vi "Super Market Billing System Edited 1.1.vi"() -> ()   [LabVIEW 2021]
uses:
  <vilib>/Utility/file.llb/Write Delimited Spreadsheet (string).vi
  <vilib>/regexp/Match Regular Expression.xnode
panel:
  in  "Tab Control":enum32{"Page 1", "Page 2", "Page 3"}(tab)
  out "Horizontal Progress Bar":u8(slide) scale=0.0..100.0
  in  "Password":string
  in  "Cashier User Name":string
  in  "OK Button":bool
  in  "Rice 5kg":bool
  in  "Dal 1kg":bool
  in  "Salt 400g":bool
  in  "Coconut Oil 1L":bool
  in  "Chilli Powder 100g":bool
  in  "Curry Powder 100g":bool
  in  "Turmeric Powder 50g":bool
  in  "Milk Powder 1kg":bool
  in  "Sugar  1kg":bool
  out "Rs.":dbl
  out "Rs.":dbl
  out "Rs.":dbl
  out "Rs.":dbl
  in  "Quantitiy":dbl min=0.0 format="%#.1f"
  out "Rs.":dbl
  in  "Quantitiy":dbl min=0.0 format="%#.1f"
  out "Rs":dbl
  in  "Quantitiy":dbl min=0.0 format="%#.1f"
  out "Rs.":dbl
  in  "Quantitiy":dbl min=0.0 format="%#.1f"
  in  "Quantitiy":dbl min=0.0 format="%#.1f"
  in  "Quantitiy":dbl min=0.0 format="%#.1f"
  in  "Quantitiy":dbl min=0.0 format="%#.1f"
  in  "Quantitiy":dbl min=0.0 format="%#.1f"
  in  "Tea 100g":bool
  in  "Quantitiy":dbl min=0.0 format="%#.1f"
  in  "Quantitiy":dbl min=0.0 format="%#.1f"
  out "Rs.":dbl
  out "Rs.":dbl
  out "Rs.":dbl
  out "Rs.":dbl
  out "Rs.":dbl
  out "Rs.":dbl
  out "Rs.":dbl
  out "Rs. 5":dbl
  out "Rs. 6":dbl
  out "Rs.":dbl
  out "Rs.":dbl
  out "Rs.":dbl
  out "Rs.":dbl
  out "Discount   Rs.":dbl format="%#.2f"
  in  "kg":dbl min=0.0 format="%#.3f"
  in  "Papaya":bool
  in  "kg":dbl min=0.0 format="%#.3f"
  in  "Graps":bool
  in  "kg":dbl min=0.0 format="%#.3f"
  in  "Orange":bool
  in  "kg":dbl min=0.0 format="%#.3f"
  in  "Apple":bool
  in  "kg":dbl min=0.0 format="%#.3f"
  in  "Banana":bool
  out "Bill   Rs.":dbl format="%#.2f"
  out "Discount percentage":string
  out "Total Bill   Rs.":dbl format="%#.2f"
  in  "kg":dbl min=0.0 format="%#.3f"
  in  "Cabege":bool
  in  "kg":dbl min=0.0 format="%#.3f"
  in  "Bringle":bool
  in  "kg":dbl min=0.0 format="%#.3f"
  in  "Beans":bool
  in  "kg":dbl min=0.0 format="%#.3f"
  in  "Leeks":bool
  in  "kg":dbl min=0.0 format="%#.3f"
  in  "Carrot":bool
  in  "stop":bool
  in  "stop 2":bool
  out "Bill Details":string
  in  "stop 3":bool
  # "WELCOME   TO  ABC                  SUPERMARCKET.."
  # "Price per 1kg (Rs.)"
  # "Quantities(kg)"
  # "Price  (Rs.)"
  # "Quantities"
  # "Fruits"
  # "Product List"
  # "Vegetables"
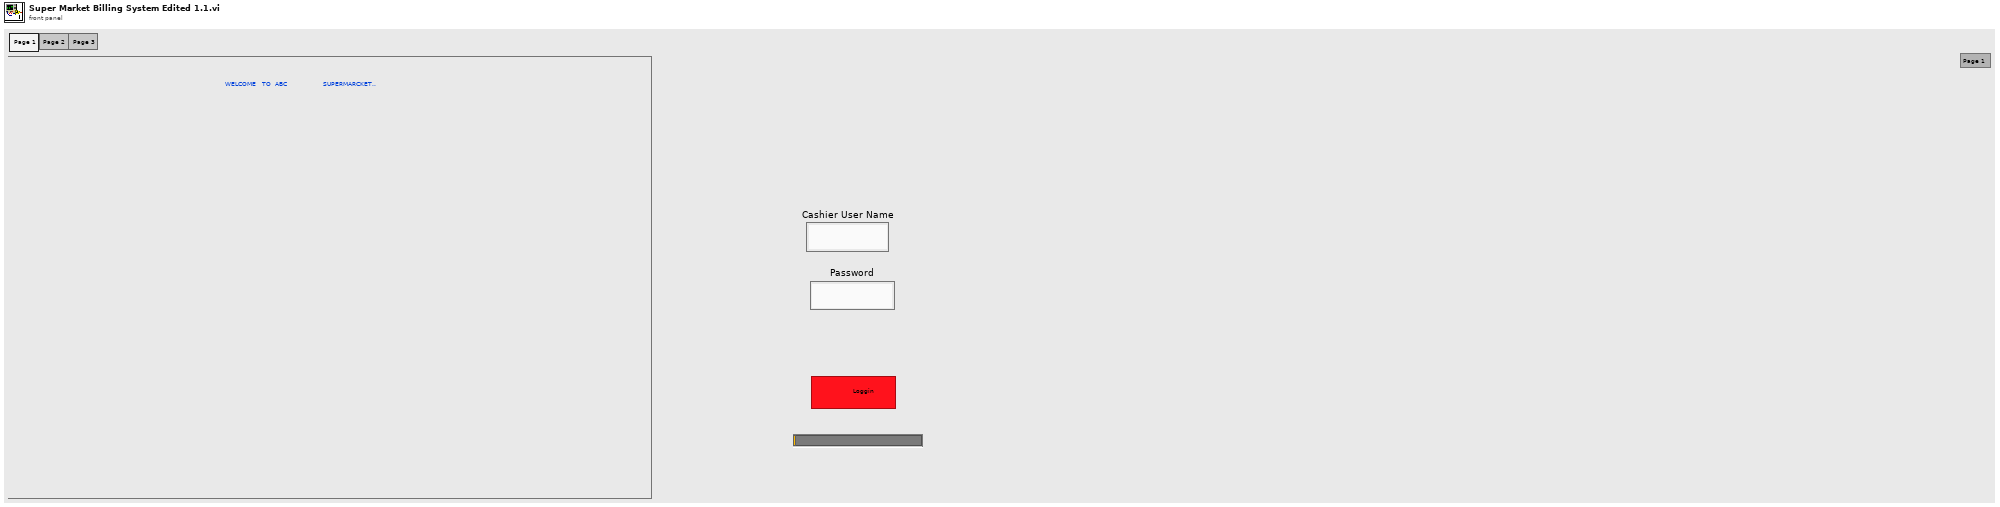
[diagram p1: front panel]
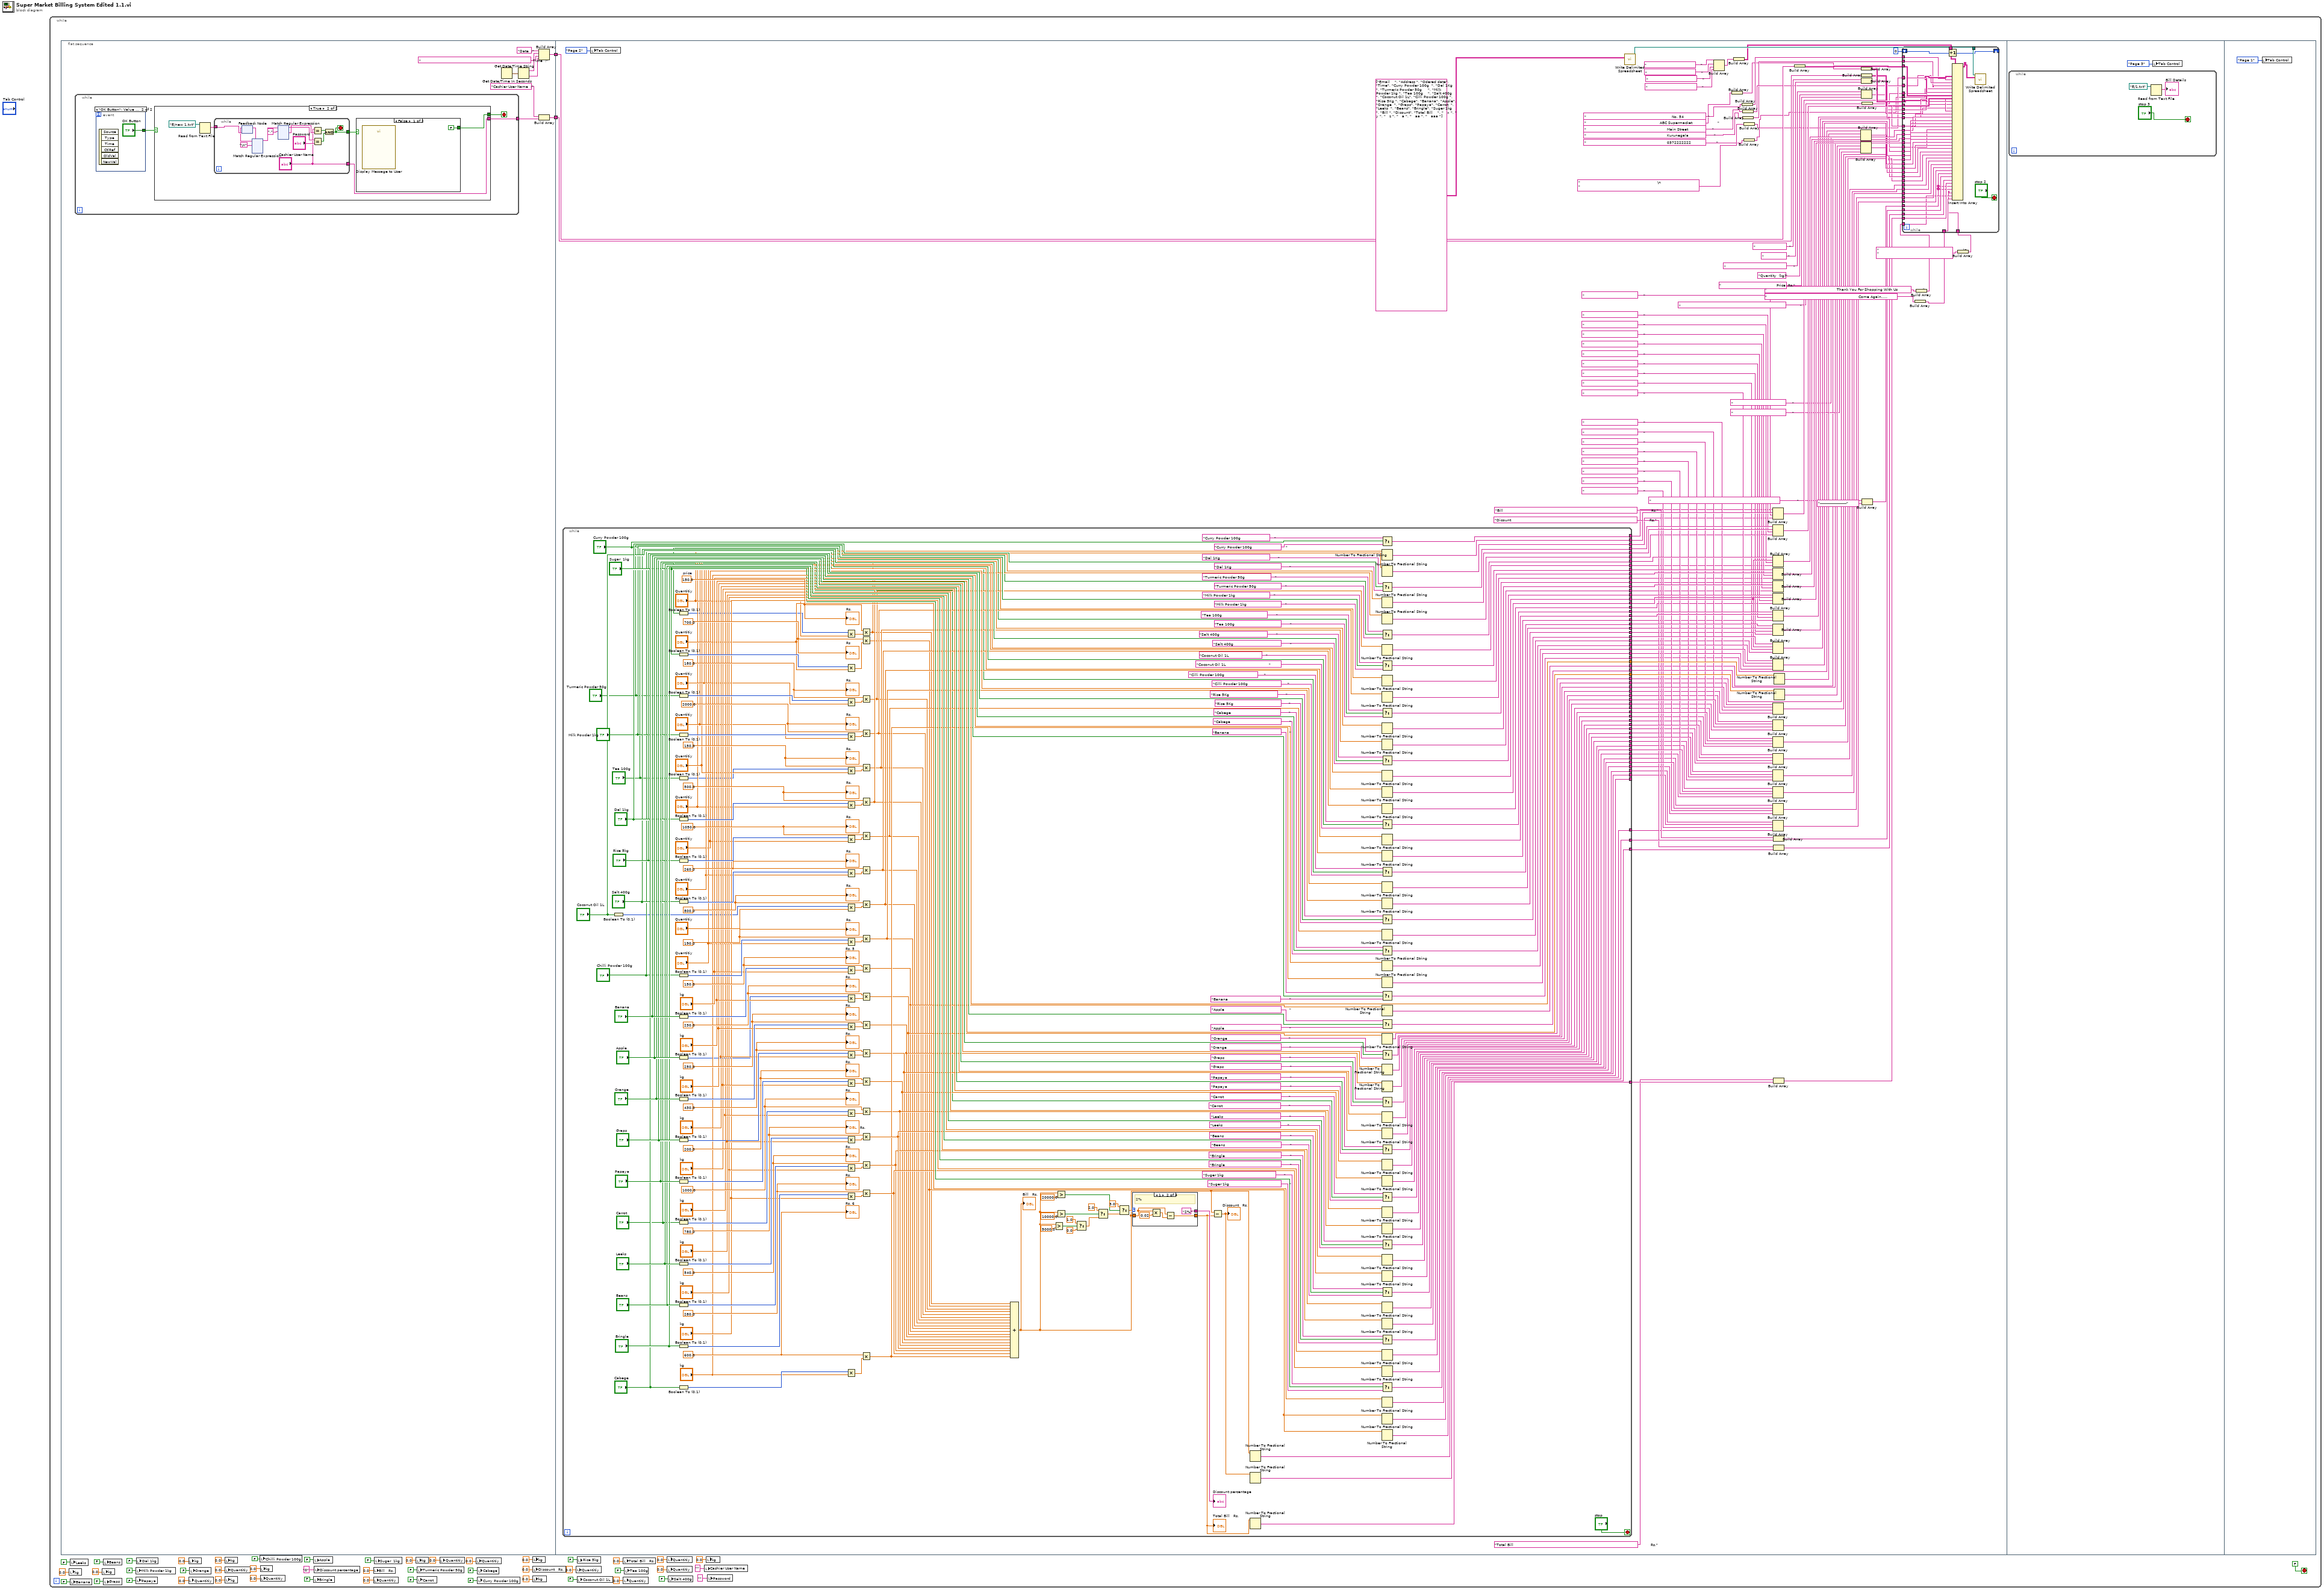
[diagram p0: block diagram]
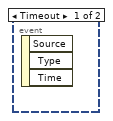
[diagram p2: hidden frame]
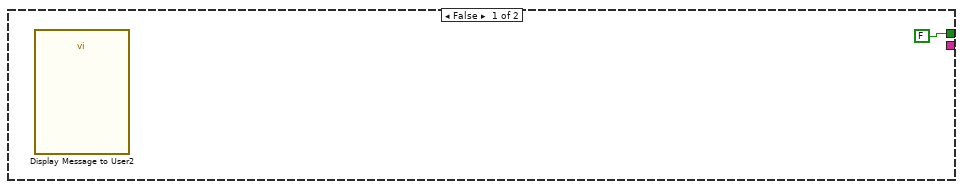
[diagram p3: hidden frame]
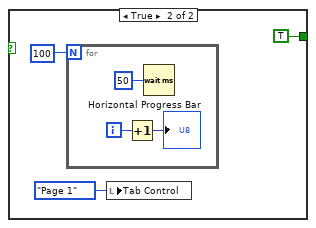
[diagram p4: hidden frame]
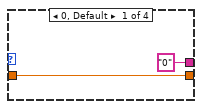
[diagram p5: hidden frame]
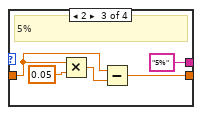
[diagram p6: hidden frame]
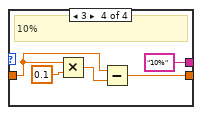
[diagram p7: hidden frame]
diagram:
  n1 = while {
    stop <- FALSE stop-if-true
    n2 = flat-sequence {
      tunnel: [w56] -> w48
      tunnel: [w52] -> w4
      tunnel: w48 -> [w351]
      tunnel: w4 -> [w418]
      frame #0 {
        n3 = while {
          tunnel: [w61] -> w50
          stop <- w60 stop-if-true
          n4 = event shown="[1] \"OK Button\": Value Change" {
            selector: _ -> [_ _]
            dyn-events: _ -> [_ _]
            timeout: _ -> [_ _]
            tunnel: [_ "OK Button"] -> w59
            event Timeout {
              n5 = event-data() -> ()  [unwired: 1 in, 3 out]
            }
            event "OK Button": Value Change {
              n6 = event-data() -> ()  [unwired: 1 in, 6 out]
            }
          }
          n7 = case shown="True" w59 {
            tunnel: [_ w66] -> w61
            tunnel: [FALSE w65] -> w60
            frame False {
              n8 = call "Display Message to User2"() -> ()  [unwired: 10 in, 2 out]
            }
            frame True {
              n9 = Read from Text File(file (use dialog)=path "E:/new 1.txt") -> (text=w68:string)  [unwired: 3 in, 3 out]
              n10 = while {
                tunnel: w68 -> [w88]
                tunnel: ["Cashier User Name"] -> w66
                tunnel: [w76] -> w64
                stop <- w76 stop-if-true
                n11 = feedback #1(w88) -> (w87:string)
                n12 = xnode "Match Regular Expression"("input string"=w87, "regular expression"="\n") -> ("before match"=w84:string, "after match"=w86:string)  [unwired: 4 in, 3 out]
                n13 = feedback-in #1(w86) -> ()
                n14 = xnode "Match Regular Expression"("input string"=w84, "regular expression"=",") -> ("before match"=w81:string, "after match"=w82:string)  [unwired: 4 in, 3 out]
                n15 = Equal?(x="Cashier User Name", y=w81) -> (x = y?=w79:bool)
                n16 = Equal?(x=w82, y="Password") -> (x = y?=w78:bool)
                n17 = And(x=w79, y=w78) -> (x .and. y?=w76:bool)
              }
              n18 = case shown="False" w64 {
                tunnel: [FALSE TRUE] -> w65
                frame False {
                  n19 = call "Display Message to User"() -> ()  [unwired: 10 in, 2 out]
                }
                frame True {
                  n20 = for {
                    N: 100 -> [_]
                    i -> [w73]
                    n21 = Increment(x=w73) -> (x+1=→"Horizontal Progress Bar":i32)
                    n22 = Wait (ms)(milliseconds to wait=u32 50 ("millisecond timer value")) -> ()  [unwired: 1 out]
                  }
                  n23 = local write "Tab Control"(enum32{"Page 1", "Page 2"}."Page 1" ("Tab Control")) -> ()
                }
              }
            }
          }
        }
        n24 = Get Date/Time In Seconds() -> (seconds since 1Jan1904=w57:timestamp)
        n25 = Get Date/Time String(seconds (now)=w57) -> (date string=w55:string, time string=w58:string)  [unwired: 2 in]
        n26 = Build Array("Date  :" ("element"), w55, "                                                                                             Time  :" ("element"), w58) -> (w56:string[])
        n27 = Build Array("Cashier User Name  :" ("element"), w50) -> (w52:string[])
      }
      frame #1 {
        n28 = while {
          tunnel: [w693] -> w471
          tunnel: [w690] -> w473
          tunnel: [w689] -> w474
          tunnel: [w681] -> w387
          tunnel: [w661] -> w441
          tunnel: [w660] -> w361
          tunnel: [w652] -> w357
          tunnel: [w651] -> w356
          tunnel: [w650] -> w355
          tunnel: [w649] -> w354
          tunnel: [w648] -> w358
          tunnel: [w647] -> w359
          tunnel: [w646] -> w432
          tunnel: ["kg"] -> w477
          tunnel: ["kg"] -> w476
          tunnel: [w642] -> w439
          tunnel: [w640] -> w438
          tunnel: [w637] -> w437
          tunnel: [w636] -> w436
          tunnel: [w635] -> w435
          tunnel: [w632] -> w434
          tunnel: [w629] -> w433
          tunnel: [w628] -> w431
          tunnel: [w601] -> w360
          tunnel: [w600] -> w333
          tunnel: [w599] -> w469
          tunnel: [w598] -> w468
          tunnel: [w597] -> w374
          tunnel: [w596] -> w465
          tunnel: [w595] -> w458
          tunnel: [w594] -> w462
          tunnel: [w593] -> w460
          tunnel: [w524] -> w459
          tunnel: [w590] -> w470
          tunnel: [w575] -> w407
          tunnel: [w588] -> w456
          tunnel: [w586] -> w467
          tunnel: [w584] -> w466
          tunnel: [w579] -> w464
          tunnel: [w522] -> w463
          tunnel: [w578] -> w461
          tunnel: [w577] -> w457
          tunnel: [w574] -> w406
          tunnel: [w573] -> w404
          tunnel: [w552] -> w402
          tunnel: [w551] -> w400
          tunnel: [w550] -> w398
          tunnel: [w548] -> w396
          tunnel: [w547] -> w394
          tunnel: [w536] -> w392
          tunnel: [w546] -> w390
          tunnel: [w545] -> w388
          tunnel: [w535] -> w385
          tunnel: [w544] -> w383
          tunnel: [w543] -> w380
          tunnel: [w542] -> w379
          tunnel: [w531] -> w377
          tunnel: [w541] -> w375
          tunnel: [w530] -> w372
          tunnel: [w540] -> w370
          tunnel: [w539] -> w368
          tunnel: [w538] -> w366
          tunnel: [w537] -> _
          stop <- "stop" stop-if-true
          w705 = 200.0 ("price")
          w702 = 430.0 ("price")
          w699 = 250.0 ("price")
          w697 = 230.0 ("price")
          w694 = 150.0 ("price")
          w720 = 600.0 ("price")
          w717 = 280.0 ("price")
          w714 = 540.0 ("price")
          w711 = 780.0 ("price")
          w708 = 1000.0 ("price")
          w747 = 150.0 ("price")
          w745 = 700.0 ("price")
          w742 = 2000.0 ("price")
          w739 = 180.0 ("price")
          w736 = 150.0  # price
          w759 = 190.0 ("price")
          w757 = 800.0 ("price")
          w754 = 260.0 ("price")
          w752 = 500.0 ("price")
          w749 = 1050.0 ("price")
          n29 = Boolean To (0,1)(Boolean="Coconut Oil 1L") -> (0, 1=w532:i16)
          n30 = Boolean To (0,1)(Boolean="Curry Powder 100g") -> (0, 1=w525:i16)
          n31 = Boolean To (0,1)(Boolean="Sugar  1kg") -> (0, 1=w746:i16)
          n32 = Boolean To (0,1)(Boolean="Turmeric Powder 50g") -> (0, 1=w740:i16)
          n33 = Boolean To (0,1)(Boolean="Milk Powder 1kg") -> (0, 1=w741:i16)
          n34 = Boolean To (0,1)(Boolean="Tea 100g") -> (0, 1=w528:i16)
          n35 = Boolean To (0,1)(Boolean="Dal 1kg") -> (0, 1=w686:i16)
          n36 = Boolean To (0,1)(Boolean="Rice 5kg") -> (0, 1=w688:i16)
          n37 = Boolean To (0,1)(Boolean="Salt 400g") -> (0, 1=w753:i16)
          n38 = Boolean To (0,1)(Boolean="Chilli Powder 100g") -> (0, 1=w687:i16)
          n39 = Boolean To (0,1)(Boolean="Banana") -> (0, 1=w685:i16)
          n40 = Boolean To (0,1)(Boolean="Apple") -> (0, 1=w534:i16)
          n41 = Boolean To (0,1)(Boolean="Orange") -> (0, 1=w698:i16)
          n42 = Boolean To (0,1)(Boolean="Graps") -> (0, 1=w703:i16)
          n43 = Boolean To (0,1)(Boolean="Papaya") -> (0, 1=w704:i16)
          n44 = Boolean To (0,1)(Boolean="Carrot") -> (0, 1=w707:i16)
          n45 = Boolean To (0,1)(Boolean="Leeks") -> (0, 1=w712:i16)
          n46 = Boolean To (0,1)(Boolean="Beans") -> (0, 1=w713:i16)
          n47 = Boolean To (0,1)(Boolean="Bringle") -> (0, 1=w718:i16)
          n48 = Boolean To (0,1)(Boolean="Cabege") -> (0, 1=w719:i16)
          n49 = Multiply(x=w525, y="Quantitiy") -> (x*y=w737:dbl)
          n50 = Multiply(x=w746, y="Quantitiy") -> (x*y=w744:dbl)
          n51 = Multiply(x=w740, y="Quantitiy") -> (x*y=w738:dbl)
          n52 = Multiply(x=w741, y="Quantitiy") -> (x*y=w743:dbl)
          n53 = Multiply(x=w528, y="Quantitiy") -> (x*y=w748:dbl)
          n54 = Multiply(x=w686, y="Quantitiy") -> (x*y=w751:dbl)
          n55 = Multiply(x=w688, y="Quantitiy") -> (x*y=w750:dbl)
          n56 = Multiply(x=w753, y="Quantitiy") -> (x*y=w755:dbl)
          n57 = Multiply(x=w532, y="Quantitiy") -> (x*y=w756:dbl)
          n58 = Multiply(x=w687, y="Quantitiy") -> (x*y=w760:dbl)
          n59 = Multiply(x=w685, y="kg") -> (x*y=w695:dbl)
          n60 = Multiply(x=w534, y="kg") -> (x*y=w696:dbl)
          n61 = Multiply(x=w698, y="kg") -> (x*y=w700:dbl)
          n62 = Multiply(x=w703, y="kg") -> (x*y=w701:dbl)
          n63 = Multiply(x=w704, y="kg") -> (x*y=w706:dbl)
          n64 = Multiply(x=w707, y="kg") -> (x*y=w709:dbl)
          n65 = Multiply(x=w712, y="kg") -> (x*y=w710:dbl)
          n66 = Multiply(x=w713, y="kg") -> (x*y=w715:dbl)
          n67 = Multiply(x=w718, y="kg") -> (x*y=w716:dbl)
          n68 = Multiply(x=w719, y="kg") -> (x*y=w721:dbl)
          n69 = Multiply(x=w736, y=w737) -> (x*y=w526:dbl)
          n70 = Multiply(x=w745, y=w744) -> (x*y=w553:dbl)
          n71 = Multiply(x=w739, y=w738) -> (x*y=w555:dbl)
          n72 = Multiply(x=w742, y=w743) -> (x*y=w556:dbl)
          n73 = Multiply(x=w747, y=w748) -> (x*y=w557:dbl)
          n74 = Multiply(x=w752, y=w751) -> (x*y=w559:dbl)
          n75 = Multiply(x=w749, y=w750) -> (x*y=w558:dbl)
          n76 = Multiply(x=w754, y=w755) -> (x*y=w560:dbl)
          n77 = Multiply(x=w757, y=w756) -> (x*y=w561:dbl)
          n78 = Multiply(x=w759, y=w760) -> (x*y=w562:dbl)
          n79 = Multiply(x=w694, y=w695) -> (x*y=w563:dbl)
          n80 = Multiply(x=w697, y=w696) -> (x*y=w564:dbl)
          n81 = Multiply(x=w699, y=w700) -> (x*y=w565:dbl)
          n82 = Multiply(x=w702, y=w701) -> (x*y=w566:dbl)
          n83 = Multiply(x=w705, y=w706) -> (x*y=w567:dbl)
          n84 = Multiply(x=w708, y=w709) -> (x*y=w568:dbl)
          n85 = Multiply(x=w711, y=w710) -> (x*y=w571:dbl)
          n86 = Multiply(x=w714, y=w715) -> (x*y=w570:dbl)
          n87 = Multiply(x=w717, y=w716) -> (x*y=w572:dbl)
          n88 = Multiply(x=w720, y=w721) -> (x*y=w569:dbl)
          n89 = Compound Arithmetic op=ADD(w526, w553, w555, w556, w557, w559, w558, w560, w561, w562, w563, w564, w565, w566, w567, w568, w571, w570, w572, w569) -> (w554:dbl)
          "Bill   Rs." <- w554
          n90 = Greater?(x=w554, y=5000.0) -> (0:w733:bool)
          n91 = Greater?(x=w554, y=20000.0) -> (0:w735:bool)
          n92 = Greater?(x=w554, y=10000.0) -> (0:w734:bool)
          n93 = Select(t=1.0, s=w733, f=0.0) -> (s? t:f=w729:dbl)
          n94 = Select(t=2.0, s=w734, f=w729) -> (s? t:f=w730:dbl)
          n95 = Select(t=3.0, s=w735, f=w730) -> (s? t:f=w731:dbl)
          n96 = case shown="1" w731 {
            tunnel: [w762 w766 w769 w774] -> w692
            tunnel: w554 -> [w762 w765 w770 w775]
            tunnel: ["0" ("discount") "2%" ("discount") "5%" ("discount") "10%" ("discount")] -> w732
            frame 0, Default {
            }
            frame 1 {
              # "2%"
              n97 = Multiply(x=w765, y=0.02) -> (x*y=w763:dbl)
              n98 = Subtract(x=w765, y=w763) -> (x-y=w766:dbl)
            }
            frame 2 {
              # "5%"
              n99 = Multiply(x=w770, y=0.05) -> (x*y=w771:dbl)
              n100 = Subtract(x=w770, y=w771) -> (x-y=w769:dbl)
            }
            frame 3 {
              # "10%"
              n101 = Multiply(x=w775, y=0.1) -> (x*y=w776:dbl)
              n102 = Subtract(x=w775, y=w776) -> (x-y=w774:dbl)
            }
          }
          "Total Bill   Rs." <- w692
          "Discount percentage" <- w732
          n103 = Subtract(x=w554, y=w692) -> (x-y=w691:dbl)
          "Discount   Rs." <- w691
          n104 = Number To Fractional String(number=w554) -> (F-format string=w693:string)  [unwired: 3 in]
          n105 = Number To Fractional String(number=w691) -> (F-format string=w689:string)  [unwired: 3 in]
          n106 = Number To Fractional String(number=w692) -> (F-format string=w690:string)  [unwired: 3 in]
          n107 = Select(t="Curry Powder 100g                            ", s="Curry Powder 100g", f="Curry Powder 100g                            ") -> (s? t:f=w600:string)
          n108 = Number To Fractional String(number="Quantitiy") -> (F-format string=w590:string)  [unwired: 3 in]
          n109 = Number To Fractional String(number=w526) -> (F-format string=w538:string)  [unwired: 3 in]
          n110 = Select(t="Dal 1Kg                                                ", s="Dal 1kg", f="Dal 1Kg                                                ") -> (s? t:f=w524:string)
          n111 = Number To Fractional String(number="Quantitiy") -> (F-format string=w577:string)  [unwired: 3 in]
          n112 = Number To Fractional String(number=w559) -> (F-format string=w531:string)  [unwired: 3 in]
          n113 = Select(t="Turmeric Powder 50g                         ", s="Turmeric Powder 50g", f="Turmeric Powder 50g                        ") -> (s? t:f=w599:string)
          n114 = Number To Fractional String(number=w555) -> (F-format string=w539:string)  [unwired: 3 in]
          n115 = Select(t="Milk Powder 1kg                                ", s="Milk Powder 1kg", f="Milk Powder 1kg                                ") -> (s? t:f=w598:string)
          n116 = Number To Fractional String(number="Quantitiy") -> (F-format string=w586:string)  [unwired: 3 in]
          n117 = Number To Fractional String(number=w556) -> (F-format string=w540:string)  [unwired: 3 in]
          n118 = Select(t="Tea 100g                                             ", s="Tea 100g", f="Tea 100g                                              ") -> (s? t:f=w597:string)
          n119 = Number To Fractional String(number="Quantitiy") -> (F-format string=w584:string)  [unwired: 3 in]
          n120 = Number To Fractional String(number=w557) -> (F-format string=w530:string)  [unwired: 3 in]
          n121 = Select(t="Salt 400g                                               ", s="Salt 400g", f="Salt 400g                                               ") -> (s? t:f=w596:string)
          n122 = Number To Fractional String(number="Quantitiy") -> (F-format string=w588:string)  [unwired: 3 in]
          n123 = Number To Fractional String(number="Quantitiy") -> (F-format string=w579:string)  [unwired: 3 in]
          n124 = Number To Fractional String(number=w560) -> (F-format string=w542:string)  [unwired: 3 in]
          n125 = Select(t="Coconut Oil 1L                               ", s="Coconut Oil 1L", f="Coconut Oil 1L                                    ") -> (s? t:f=w595:string)
          n126 = Number To Fractional String(number="Quantitiy") -> (F-format string=w522:string)  [unwired: 3 in]
          n127 = Number To Fractional String(number=w561) -> (F-format string=w543:string)  [unwired: 3 in]
          n128 = Select(t="Cilli Powder 100g                                 ", s="Chilli Powder 100g", f="Cilli Powder 100g                                 ") -> (s? t:f=w594:string)
          n129 = Number To Fractional String(number="Quantitiy") -> (F-format string=w578:string)  [unwired: 3 in]
          n130 = Number To Fractional String(number=w562) -> (F-format string=w544:string)  [unwired: 3 in]
          n131 = Select(t="Rise 5Kg                                               ", s="Rice 5kg", f="Rise 5Kg                                              ") -> (s? t:f=w593:string)
          n132 = Number To Fractional String(number=w558) -> (F-format string=w541:string)  [unwired: 3 in]
          n133 = Select(t="Cabege                                                ", s="Cabege", f="Cabege                                                 ") -> (s? t:f=w646:string)
          n134 = Number To Fractional String(number="kg") -> (F-format string=w628:string)  [unwired: 3 in]
          n135 = Number To Fractional String(number=w569) -> (F-format string=w552:string)  [unwired: 3 in]
          n136 = Select(t="Banana                                                  ", s="Banana", f="Banana                                                   ") -> (s? t:f=w681:string)
          n137 = Number To Fractional String(number=w563) -> (F-format string=w535:string)  [unwired: 3 in]
          n138 = Select(t="Apple                                                      ", s="Apple", f="Apple                                                      ") -> (s? t:f=w661:string)
          n139 = Number To Fractional String(number=w564) -> (F-format string=w545:string)  [unwired: 3 in]
          n140 = Select(t="Orange                                                   ", s="Orange", f="Orange                                                    ") -> (s? t:f=w660:string)
          n141 = Number To Fractional String(number="kg") -> (F-format string=w642:string)  [unwired: 3 in]
          n142 = Number To Fractional String(number=w565) -> (F-format string=w546:string)  [unwired: 3 in]
          n143 = Select(t="Graps                                                      " ("f"), s="Graps", f="Graps                                                       ") -> (s? t:f=w652:string)
          n144 = Number To Fractional String(number="kg") -> (F-format string=w640:string)  [unwired: 3 in]
          n145 = Number To Fractional String(number=w566) -> (F-format string=w536:string)  [unwired: 3 in]
          n146 = Select(t="Papaya                                                    ", s="Papaya", f="Papaya                                                    ") -> (s? t:f=w651:string)
          n147 = Number To Fractional String(number="kg") -> (F-format string=w637:string)  [unwired: 3 in]
          n148 = Number To Fractional String(number=w567) -> (F-format string=w547:string)  [unwired: 3 in]
          n149 = Select(t="Carrot                                                      ", s="Carrot", f="Carrot                                                       ") -> (s? t:f=w650:string)
          n150 = Number To Fractional String(number="kg") -> (F-format string=w636:string)  [unwired: 3 in]
          n151 = Number To Fractional String(number=w568) -> (F-format string=w548:string)  [unwired: 3 in]
          n152 = Select(t="Leeks                                                       ", s="Leeks", f="Leeks                                                      ") -> (s? t:f=w649:string)
          n153 = Number To Fractional String(number="kg") -> (F-format string=w635:string)  [unwired: 3 in]
          n154 = Number To Fractional String(number=w571) -> (F-format string=w550:string)  [unwired: 3 in]
          n155 = Select(t="Beans                                                       ", s="Beans", f="Beans                                                      ") -> (s? t:f=w648:string)
          n156 = Number To Fractional String(number="kg") -> (F-format string=w632:string)  [unwired: 3 in]
          n157 = Number To Fractional String(number=w570) -> (F-format string=w551:string)  [unwired: 3 in]
          n158 = Select(t="Bringle                                                      ", s="Bringle", f="Bringle                                                      ") -> (s? t:f=w647:string)
          n159 = Number To Fractional String(number="kg") -> (F-format string=w629:string)  [unwired: 3 in]
          n160 = Number To Fractional String(number=w572) -> (F-format string=w573:string)  [unwired: 3 in]
          n161 = Select(t="Suger 1kg                                                  ", s="Sugar  1kg", f="Suger 1kg                                                  ") -> (s? t:f=w601:string)
          n162 = Number To Fractional String(number="Quantitiy") -> (F-format string=w575:string)  [unwired: 3 in]
          n163 = Number To Fractional String(number=w553) -> (F-format string=w537:string)  [unwired: 3 in]
          n164 = Number To Fractional String(number=w553) -> (F-format string=w574:string)  [unwired: 3 in]
          "Rs." <- w749
          "Rs." <- w752
          "Rs." <- w754
          "Rs." <- w757
          "Rs." <- w759
          "Rs." <- w736
          "Rs." <- w739
          "Rs." <- w742
          "Rs" <- w745
          "Rs." <- w747
          "Rs." <- w708
          "Rs." <- w711
          "Rs." <- w714
          "Rs." <- w717
          "Rs. 6" <- w720
          "Rs. 5" <- w694
          "Rs." <- w697
          "Rs." <- w699
          "Rs." <- w702
          "Rs." <- w705
        }
        n165 = local write "Tab Control"(enum32{"Page 1", "Page 2"}."Page 2" ("Tab Control")) -> ()
        n166 = call-poly <vilib>:"Write Delimited Spreadsheet.vi"("2D data"=string[][] [["Email    "], ["Address "], ["Odered date"], ["Time"], ["Curry Powder 100g  "], ["Dal 1Kg   "], ["Turmeric Powder 50g     "], ["Milk Powder 1kg "], ["Tea 100g    "], ["Salt 400g   "], ["Coconut Oil 1L"], ["Cilli Powder 100g "], ["Rise 5Kg "], ["Cabege"], ["Banana"], ["Apple"], ["Orange  "], ["Graps"], ["Papaya"], ["Carrot  "], ["Leeks  "], ["Beans"], ["Bringle"], ["Suger 1kg  "], ["Bill "], ["Dicount"], ["Total Bill    "], ["   x "], ["   y "], ["   z "], ["   a "], ["   aa "], ["   aaa "]] ("delimiter (\\t)")) -> ("new file path (Not A Path if cancelled)"=w352:path)  [unwired: 13 in, 1 out]
        n167 = Build Array("                                             ", "                                             ", "                                             ", "                                             ") -> (w342:string[])
        n168 = Build Array("                                                             ABC Supermacket                     ") -> (w329:string[])
        n169 = Build Array(w342) -> (w337:string[][])
        n170 = Build Array("                                                                       No. 54                    ") -> (w346:string[])
        n171 = Build Array("                                                                   Main Street                    ") -> (w345:string[])
        n172 = Build Array("                                                                   Kurunegala                     ") -> (w344:string[])
        n173 = Build Array("                                                                   0372222222                     ") -> (w327:string[])
        n174 = Build Array("                                                                \n                                                ") -> (w343:string[])
        n175 = Build Array(w333, w470, "                                                 " ("element"), w366) -> (w451:string[])
        n176 = Build Array(w459, w457, "                                                 " ("element"), w377) -> (w443:string[])
        n177 = Build Array(w469, w456, "                                                 " ("element"), w368) -> (w450:string[])
        n178 = Build Array(w468, w467, "                                                 " ("element"), w370) -> (w449:string[])
        n179 = Build Array(w374, w466, "                                                 " ("element"), w372) -> (w448:string[])
        n180 = Build Array(w465, w464, "                                                 " ("element"), w379) -> (w447:string[])
        n181 = Build Array(w458, w463, "                                                 " ("element"), w380) -> (w446:string[])
        n182 = Build Array(w462, w461, "                                                 " ("element"), w383) -> (w445:string[])
        n183 = Build Array(w460, w456, "                                                 " ("element"), w375) -> (w444:string[])
        n184 = Build Array(w432, w431, "                                                 " ("element"), w402) -> (w421:string[])
        n185 = Build Array(w361, w439, "                                                 " ("element"), w390) -> (w428:string[])
        n186 = Build Array(w357, w438, "                                                 " ("element"), w392) -> (w427:string[])
        n187 = Build Array(w356, w437, "                                                 " ("element"), w394) -> (w426:string[])
        n188 = Build Array(w355, w436, "                                                 " ("element"), w396) -> (w425:string[])
        n189 = Build Array(w354, w435, "                                                 " ("element"), w398) -> (w424:string[])
        n190 = Build Array(w358, w434, "                                                 " ("element"), w400) -> (w423:string[])
        n191 = Build Array(w359, w433, "                                                 " ("element"), w404) -> (w422:string[])
        n192 = Build Array(w360, w407, "                                                 " ("element"), w406) -> (w452:string[])
        n193 = Build Array("Bill                                                                                                                           Rs." ("element"), w471) -> (w454:string[])
        n194 = Build Array("Dicount                                                                                                                   Rs." ("element"), w474) -> (w409:string[])
        n195 = Build Array("Total Bill                                                                                                                  Rs." ("element"), w473) -> (w453:string[])
        n196 = Number To Fractional String(number=w477) -> (F-format string=w442:string)  [unwired: 3 in]
        n197 = Number To Fractional String(number=w476) -> (F-format string=w440:string)  [unwired: 3 in]
        n198 = Build Array(w351) -> (w350:string[][])
        n199 = Build Array(w387, w442, "                                                 " ("element"), w385) -> (w430:string[])
        n200 = Build Array(w441, w440, "                                                 " ("element"), w388) -> (w429:string[])
        n201 = Build Array("                                                        " ("element"), "Quantity  (kg)" ("element"), "                                              Price  Rs." ("element")) -> (w411:string[])
        n202 = Build Array(w329) -> (w455:string[][])
        n203 = Build Array(w418) -> (w417:string[][])
        n204 = Build Array("                            ", "                    " ("element")) -> (w413:string[])
        n205 = Build Array("                                                                                                   ") -> (w332:string[])
        n206 = Build Array("                                                                                                                         ", "----------------------" ("element")) -> (w364:string[])
        n207 = Build Array("                                                                            Come Again.....                     " ("element")) -> (w325:string[])
        n208 = Build Array("                                                          Thank You For Shopping With Us                     " ("element")) -> (w331:string[])
        n209 = Build Array("                                                                      \n                                                     " ("element")) -> (w323:string[])
        n210 = while {
          tunnel: w352 -> [w521]
          shift-right: [w518] -> _
          shift-left: 0 -> [w519]
          tunnel: w455 -> [w486]
          tunnel: w454 -> [w496]
          tunnel: w409 -> [w495]
          tunnel: w453 -> [w494]
          tunnel: w452 -> [w497]
          tunnel: w451 -> [w489]
          tunnel: w450 -> [w500]
          tunnel: w449 -> [w501]
          tunnel: w448 -> [w502]
          tunnel: w447 -> [w503]
          tunnel: w446 -> [w504]
          tunnel: w445 -> [w505]
          tunnel: w444 -> [w506]
          tunnel: w443 -> [w499]
          tunnel: w430 -> [w508]
          tunnel: w429 -> [w509]
          tunnel: w428 -> [w510]
          tunnel: w427 -> [w511]
          tunnel: w426 -> [w512]
          tunnel: w425 -> [w513]
          tunnel: w424 -> [w514]
          tunnel: w423 -> [w515]
          tunnel: w422 -> [w516]
          tunnel: w421 -> [w507]
          tunnel: w417 -> [w517]
          tunnel: w413 -> [w498]
          tunnel: w411 -> [w488]
          tunnel: w364 -> [w478]
          tunnel: w350 -> [w492]
          tunnel: w346 -> [w485]
          tunnel: w345 -> [w484]
          tunnel: w344 -> [w483]
          tunnel: w343 -> [w491]
          tunnel: w337 -> [w490]
          tunnel: w332 -> [w487]
          tunnel: w331 -> [w480]
          tunnel: w327 -> [w482]
          tunnel: w325 -> [w481]
          tunnel: w323 -> [w479]
          stop <- "stop 2" stop-if-true
          n211 = Increment(x=w519) -> (x+1=w518:i32)
          n212 = Insert Into Array(array=w490, new element #1=w486, new element #2=w485, new element #3=w484, new element #4=w483, new element #5=w482, new element #6=w491, new element #7=w492, new element #8=w517, new element #9=w498, new element #10=w487, new element #11=w488, new element #12=w489, new element #13=w499, new element #14=w500, new element #15=w501, new element #16=w502, new element #17=w503, new element #18=w504, new element #19=w505, new element #20=w506, new element #21=w507, new element #22=w508, new element #23=w509, new element #24=w510, new element #25=w511, new element #26=w512, new element #27=w513, new element #28=w514, new element #29=w515, new element #30=w516, new element #31=w497, new element #32=w478, new element #33=w496, new element #34=w495, new element #35=w494, new element #36=w478, new element #37=w478, new element #38=w479, new element #39=w480, new element #40=w481) -> (w493:string[][])  [unwired: 2 in]
          n213 = call-poly <vilib>:"Write Delimited Spreadsheet.vi"("file path (dialog if empty)"=w521, "2D data"=w493) -> ()  [unwired: 12 in, 2 out]
        }
      }
      frame #2 {
        n214 = while {
          stop <- "stop 3" stop-if-true
          n215 = Read from Text File(file (use dialog)=path "E:/1.txt") -> (text=→"Bill Details":string)  [unwired: 3 in, 3 out]
        }
        n216 = local write "Tab Control"(enum32{"Page 1", "Page 2", "Page 3"}."Page 3" ("Tab Control")) -> ()
      }
      frame #3 {
        n217 = local write "Tab Control"(enum32{"Page 1", "Page 2"}."Page 1" ("Tab Control")) -> ()
      }
    }
    n218 = local write "kg"(0.0 ("kg")) -> ()
    n219 = local write "Leeks"(FALSE ("Leeks")) -> ()
    n220 = local write "Banana"(FALSE ("Banana")) -> ()
    n221 = local write "kg"(0.0 ("kg")) -> ()
    n222 = local write "Beans"(FALSE ("Beans")) -> ()
    n223 = local write "Graps"(FALSE ("Graps")) -> ()
    n224 = local write "Milk Powder 1kg"(FALSE ("Milk Powder 1kg")) -> ()
    n225 = local write "Papaya"(FALSE ("Papaya")) -> ()
    n226 = local write "Dal 1kg"(FALSE ("Dal 1Kg")) -> ()
    n227 = local write "kg"(0.0 ("kg")) -> ()
    n228 = local write "Quantitiy"(0.0 ("Quantities")) -> ()
    n229 = local write "Orange"(FALSE ("Orange")) -> ()
    n230 = local write "kg"(0.0 ("kg")) -> ()
    n231 = local write "Quantitiy"(0.0 ("quantity 15")) -> ()
    n232 = local write "kg"(0.0 ("kg")) -> ()
    n233 = local write "Chilli Powder 100g"(FALSE ("Cilli Powder 100g")) -> ()
    n234 = local write "kg"(0.0 ("kg")) -> ()
    n235 = local write "Quantitiy"(0.0 ("quantity 17")) -> ()
    n236 = local write "Apple"(FALSE ("Apple")) -> ()
    n237 = local write "Bringle"(FALSE ("Bringle")) -> ()
    n238 = local write "Discount percentage"("0" ("Discount percentage")) -> ()
    n239 = local write "Bill   Rs."(0.0 ("Bill   Rs.")) -> ()
    n240 = local write "Quantitiy"(0.0 ("quantity 10")) -> ()
    n241 = local write "Sugar  1kg"(FALSE ("Sugar  1kg")) -> ()
    n242 = local write "kg"(0.0 ("kg")) -> ()
    n243 = local write "Turmeric Powder 50g"(FALSE ("Turmeric Powder 50g")) -> ()
    n244 = local write "Carrot"(FALSE ("Carrot")) -> ()
    n245 = local write "Quantitiy"(0.0 ("quantity 16")) -> ()
    n246 = local write "Quantitiy"(0.0 ("quantity 12")) -> ()
    n247 = local write "Cabege"(FALSE ("Cabege")) -> ()
    n248 = local write "Curry Powder 100g"(FALSE ("Curry Powder 100g")) -> ()
    n249 = local write "kg"(0.0 ("kg")) -> ()
    n250 = local write "Discount   Rs."(0.0 ("Discount   Rs.")) -> ()
    n251 = local write "kg"(0.0 ("kg")) -> ()
    n252 = local write "Quantitiy"(0.0 ("quantity 13")) -> ()
    n253 = local write "Rice 5kg"(FALSE ("Rise 5Kg")) -> ()
    n254 = local write "Coconut Oil 1L"(FALSE ("Coconut Oil 1L")) -> ()
    n255 = local write "Total Bill   Rs."(0.0 ("Total Bill   Rs.")) -> ()
    n256 = local write "Quantitiy"(0.0 ("quantity 14")) -> ()
    n257 = local write "Tea 100g"(FALSE ("Tea 100g")) -> ()
    n258 = local write "Quantitiy"(0.0 ("quantity 11")) -> ()
    n259 = local write "Quantitiy"(0.0 ("Quantities 4")) -> ()
    n260 = local write "Salt 400g"(FALSE ("Salt 400g")) -> ()
    n261 = local write "Cashier User Name"("" ("String")) -> ()
    n262 = local write "kg"(0.0 ("kg")) -> ()
    n263 = local write "Password"("" ("String 2")) -> ()
  }
